vi "Main Test.vi"() -> ()   [LabVIEW 2020]
uses:
  Mete.ctl
  R.ctl
  P.ctl
  N.ctl
  D.ctl
  Odo Velocity.ctl
  Gas.ctl
  Set-.ctl
  Set+.ctl
  Cru.ctl
  Dis.ctl
  CharRPM.ctl
  Brake.ctl
  Limit.ctl
  SET+LIMIT.ctl
  SET-LIMIT.ctl
  CharODO.ctl
  STOP.ctl
  ssas.ctl
  indicator.ctl
  Volum MODE.ctl
panel:
  in  "Cruise control Mode":T1=1 scale=1.0..3.0
  out "Numeric":T2
  in  "Tab Control":T3
  out "Image":T4(plugin-control)
  out "Boolean":T5
  in  "LIMIT-":T6
  in  "LIMT+":T7
  in  "LIMIT":T8
  in  "Slide 4":T9 scale=0.0..700.0
  out "Waveform Chart":T10
  out "Waveform Chart 2":T11
  in  "Dis":T12 caption="Boolean 8"
  in  "Cu":T13 caption="Boolean 7"
  in  "+Cu":T14 caption="Boolean 5"
  in  "-Cu":T15 caption="Boolean 6"
  in  "Slide 2":T16 scale=0.0..700.0
  out "Km/h":T17 scale=0.0..250.0
  in  "stop":T18
  out "Boolean 4":T19
  out "Boolean 3":T20
  out "Boolean 2":T21
  out "Gauge":T22 scale=0.0..650.0
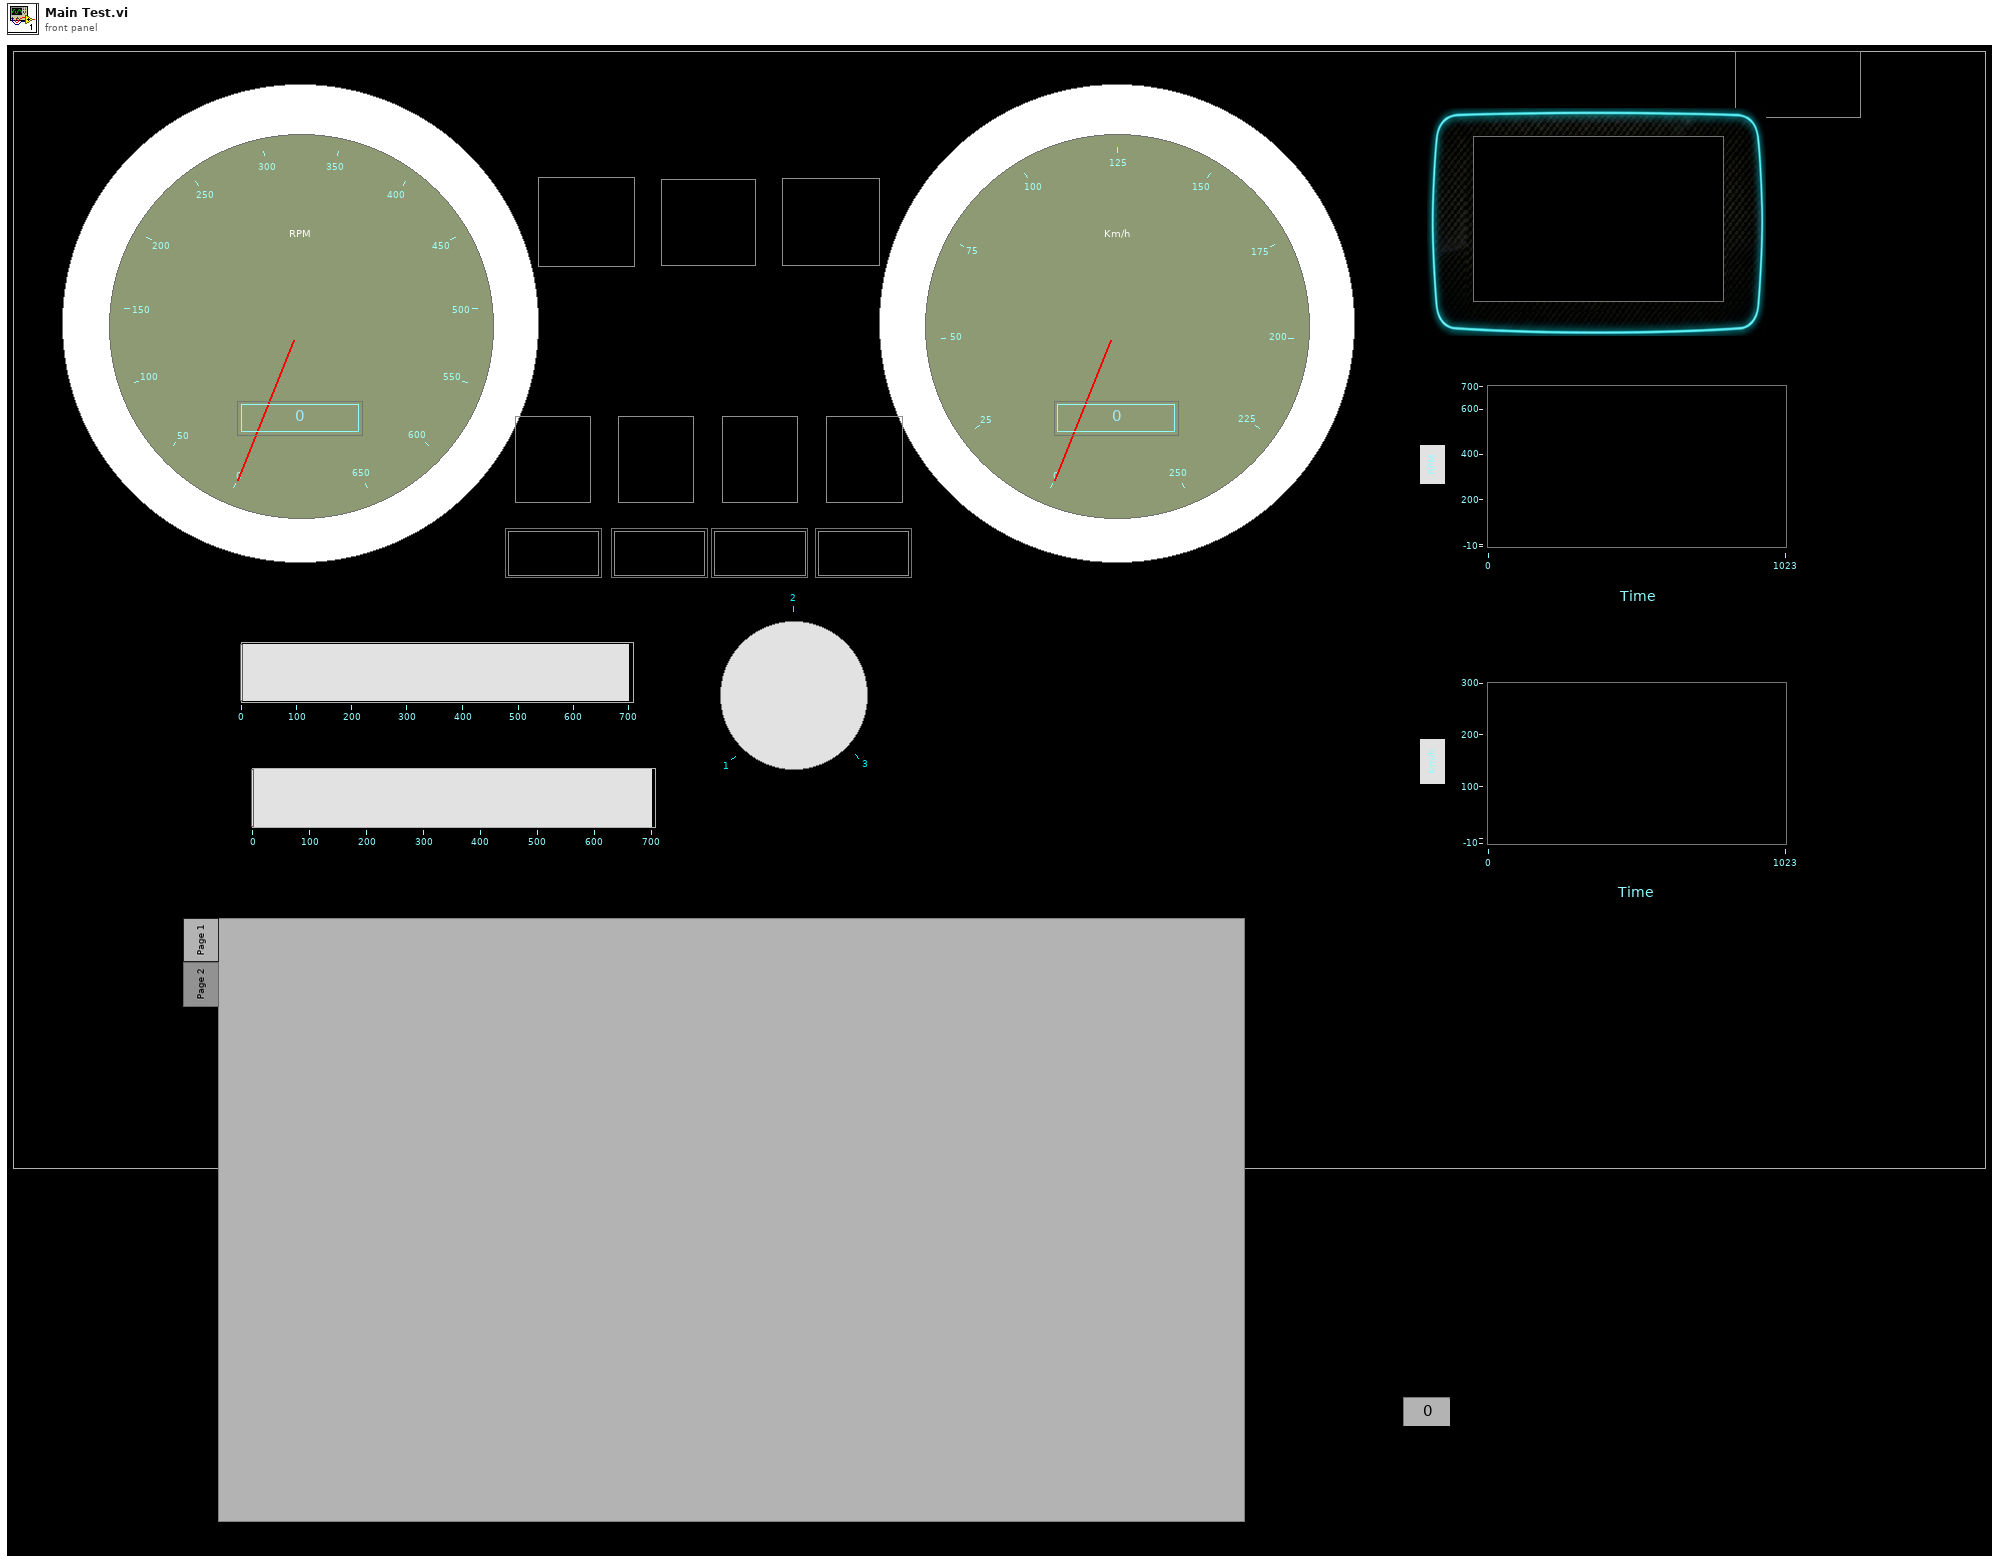
[diagram p1: front panel]
types:
  T1 = typedef "Volum MODE.ctl" = u8
  T2 = typedef "indicator.ctl" = dbl
  T3 = typedef "ssas.ctl" = enum32{"Page 1", "Page 2"}
  T4 = typedef "IMAQ Image.ctl" = refnum<image>
  T5 = typedef "R.ctl" = bool
  T6 = typedef "SET-LIMIT.ctl" = bool
  T7 = typedef "SET+LIMIT.ctl" = bool
  T8 = typedef "Limit.ctl" = bool
  T9 = typedef "Brake.ctl" = dbl
  T10 = typedef "CharODO.ctl" = dbl
  T11 = typedef "CharRPM.ctl" = dbl
  T12 = typedef "Dis.ctl" = bool
  T13 = typedef "Cru.ctl" = bool
  T14 = typedef "Set+.ctl" = bool
  T15 = typedef "Set-.ctl" = bool
  T16 = typedef "Gas.ctl" = dbl
  T17 = typedef "Odo Velocity.ctl" = u16
  T18 = typedef "STOP.ctl" = bool
  T19 = typedef "D.ctl" = bool
  T20 = typedef "N.ctl" = bool
  T21 = typedef "P.ctl" = bool
  T22 = typedef "Mete.ctl" = u16
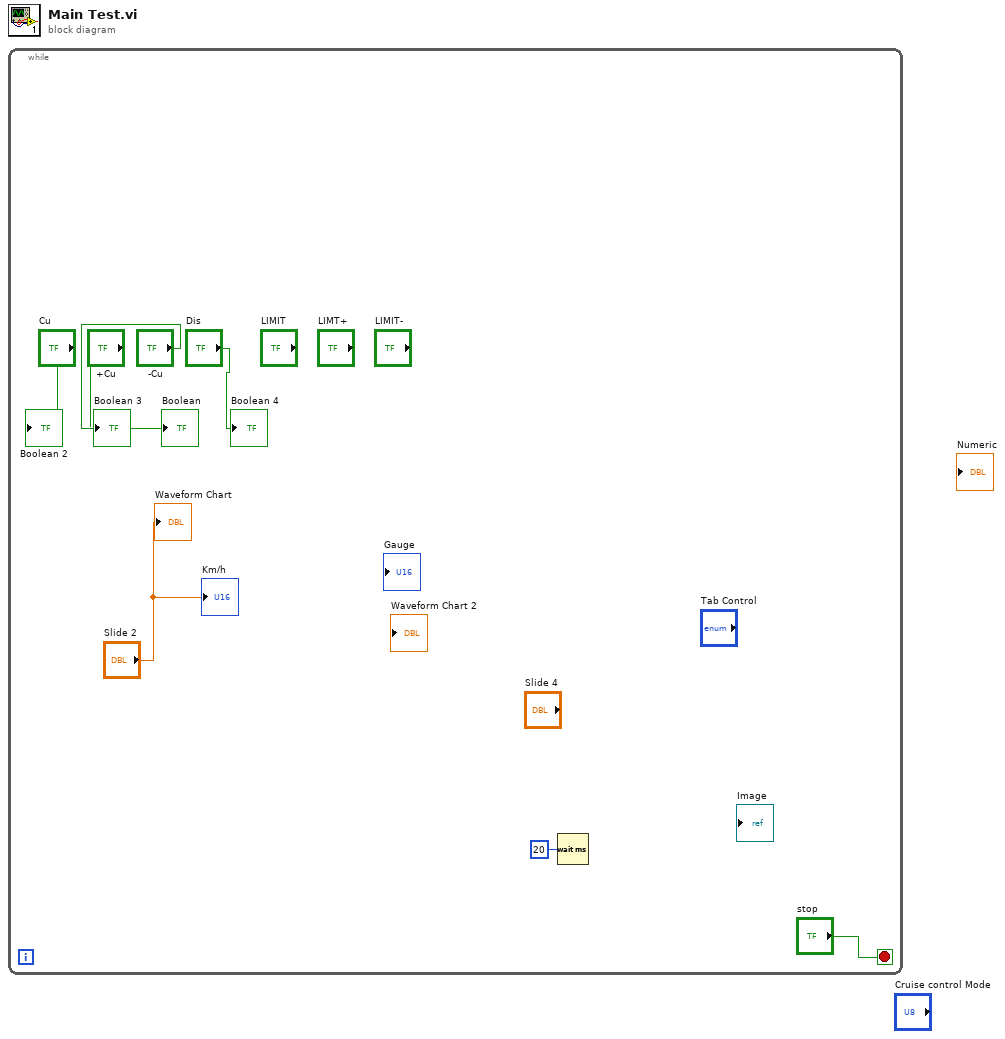
[diagram p0: block diagram]
diagram:
  n1 = while {
    stop <- "stop" stop-if-true
    n2 = Wait (ms)(milliseconds to wait=u32 20) -> ()  [unwired: 1 out]
    "Boolean 2" <- "Cu"
    "Boolean 3" <- "+Cu"
    "Boolean" <- "-Cu"
    "Boolean 4" <- "Dis"
    "Km/h" <- "Slide 2"
    "Waveform Chart" <- "Slide 2"
  }
